vi "Super Market Billing System Final output.vi"() -> ()   [LabVIEW 2021]
uses:
  <vilib>/Utility/file.llb/Write Delimited Spreadsheet (string).vi
  <vilib>/regexp/Match Regular Expression.xnode
panel:
  in  "Tab Control":enum32{"Page 1", "Page 2", "Page 3"}(tab)
  out "Horizontal Progress Bar":u8(slide) scale=0.0..100.0
  in  "Password":string
  in  "Cashier User Name":string
  in  "OK Button":bool
  in  "Rice 5kg":bool
  in  "Dal 1kg":bool
  in  "Salt 400g":bool
  in  "Coconut Oil 1L":bool
  in  "Chilli Powder 100g":bool
  in  "Curry Powder 100g":bool
  in  "Turmeric Powder 50g":bool
  in  "Milk Powder 1kg":bool
  in  "Sugar  1kg":bool
  out "Rs.":dbl
  out "Rs.":dbl
  out "Rs.":dbl
  out "Rs.":dbl
  in  "Quantitiy":dbl min=0.0 format="%#.1f"
  out "Rs.":dbl
  in  "Quantitiy":dbl min=0.0 format="%#.1f"
  out "Rs":dbl
  in  "Quantitiy":dbl min=0.0 format="%#.1f"
  out "Rs.":dbl
  in  "Quantitiy":dbl min=0.0 format="%#.1f"
  in  "Quantitiy":dbl min=0.0 format="%#.1f"
  in  "Quantitiy":dbl min=0.0 format="%#.1f"
  in  "Quantitiy":dbl min=0.0 format="%#.1f"
  in  "Quantitiy":dbl min=0.0 format="%#.1f"
  in  "Tea 100g":bool
  in  "Quantitiy":dbl min=0.0 format="%#.1f"
  in  "Quantitiy":dbl min=0.0 format="%#.1f"
  out "Rs.":dbl
  out "Rs.":dbl
  out "Rs.":dbl
  out "Rs.":dbl
  out "Rs.":dbl
  out "Rs.":dbl
  out "Rs.":dbl
  out "Rs. 5":dbl
  out "Rs. 6":dbl
  out "Rs.":dbl
  out "Rs.":dbl
  out "Rs.":dbl
  out "Rs.":dbl
  out "Discount   Rs.":dbl format="%#.2f"
  in  "kg":dbl min=0.0 format="%#.3f"
  in  "Papaya":bool
  in  "kg":dbl min=0.0 format="%#.3f"
  in  "Graps":bool
  in  "kg":dbl min=0.0 format="%#.3f"
  in  "Orange":bool
  in  "kg":dbl min=0.0 format="%#.3f"
  in  "Apple":bool
  in  "kg":dbl min=0.0 format="%#.3f"
  in  "Banana":bool
  out "Bill   Rs.":dbl format="%#.2f"
  out "Discount percentage":string
  out "Total Bill   Rs.":dbl format="%#.2f"
  in  "kg":dbl min=0.0 format="%#.3f"
  in  "Cabege":bool
  in  "kg":dbl min=0.0 format="%#.3f"
  in  "Bringle":bool
  in  "kg":dbl min=0.0 format="%#.3f"
  in  "Beans":bool
  in  "kg":dbl min=0.0 format="%#.3f"
  in  "Leeks":bool
  in  "kg":dbl min=0.0 format="%#.3f"
  in  "Carrot":bool
  in  "stop":bool
  in  "stop 2":bool
  out "Bill Details":string
  in  "stop 3":bool
  # "WELCOME   TO  ABC                  SUPERMARCKET.."
  # "Price per 1kg (Rs.)"
  # "Quantities(kg)"
  # "Price  (Rs.)"
  # "Quantities"
  # "Fruits"
  # "Product List"
  # "Vegetables"
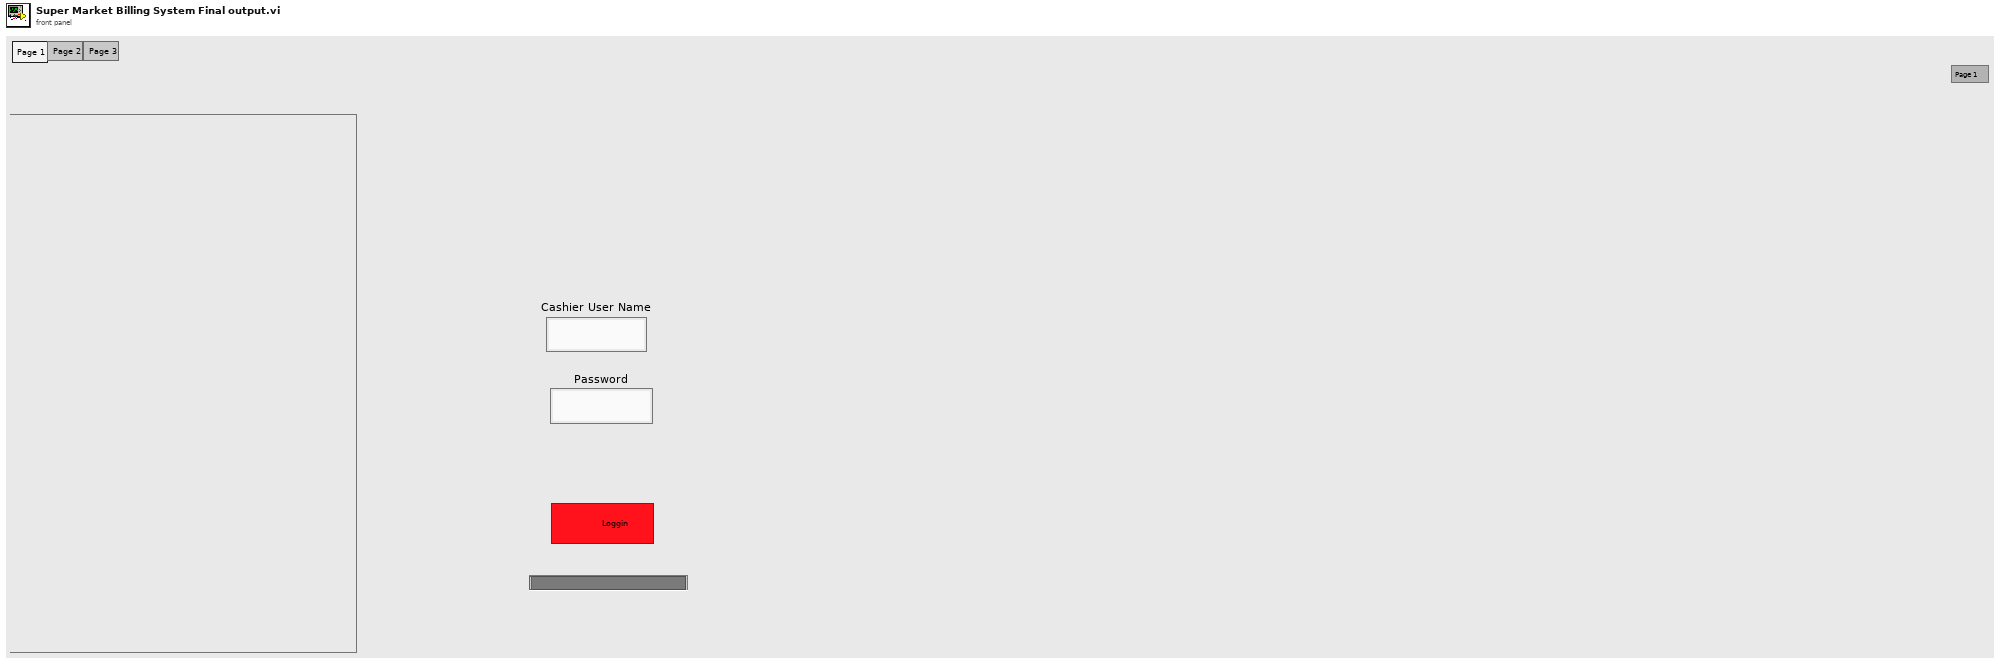
[diagram p1: front panel]
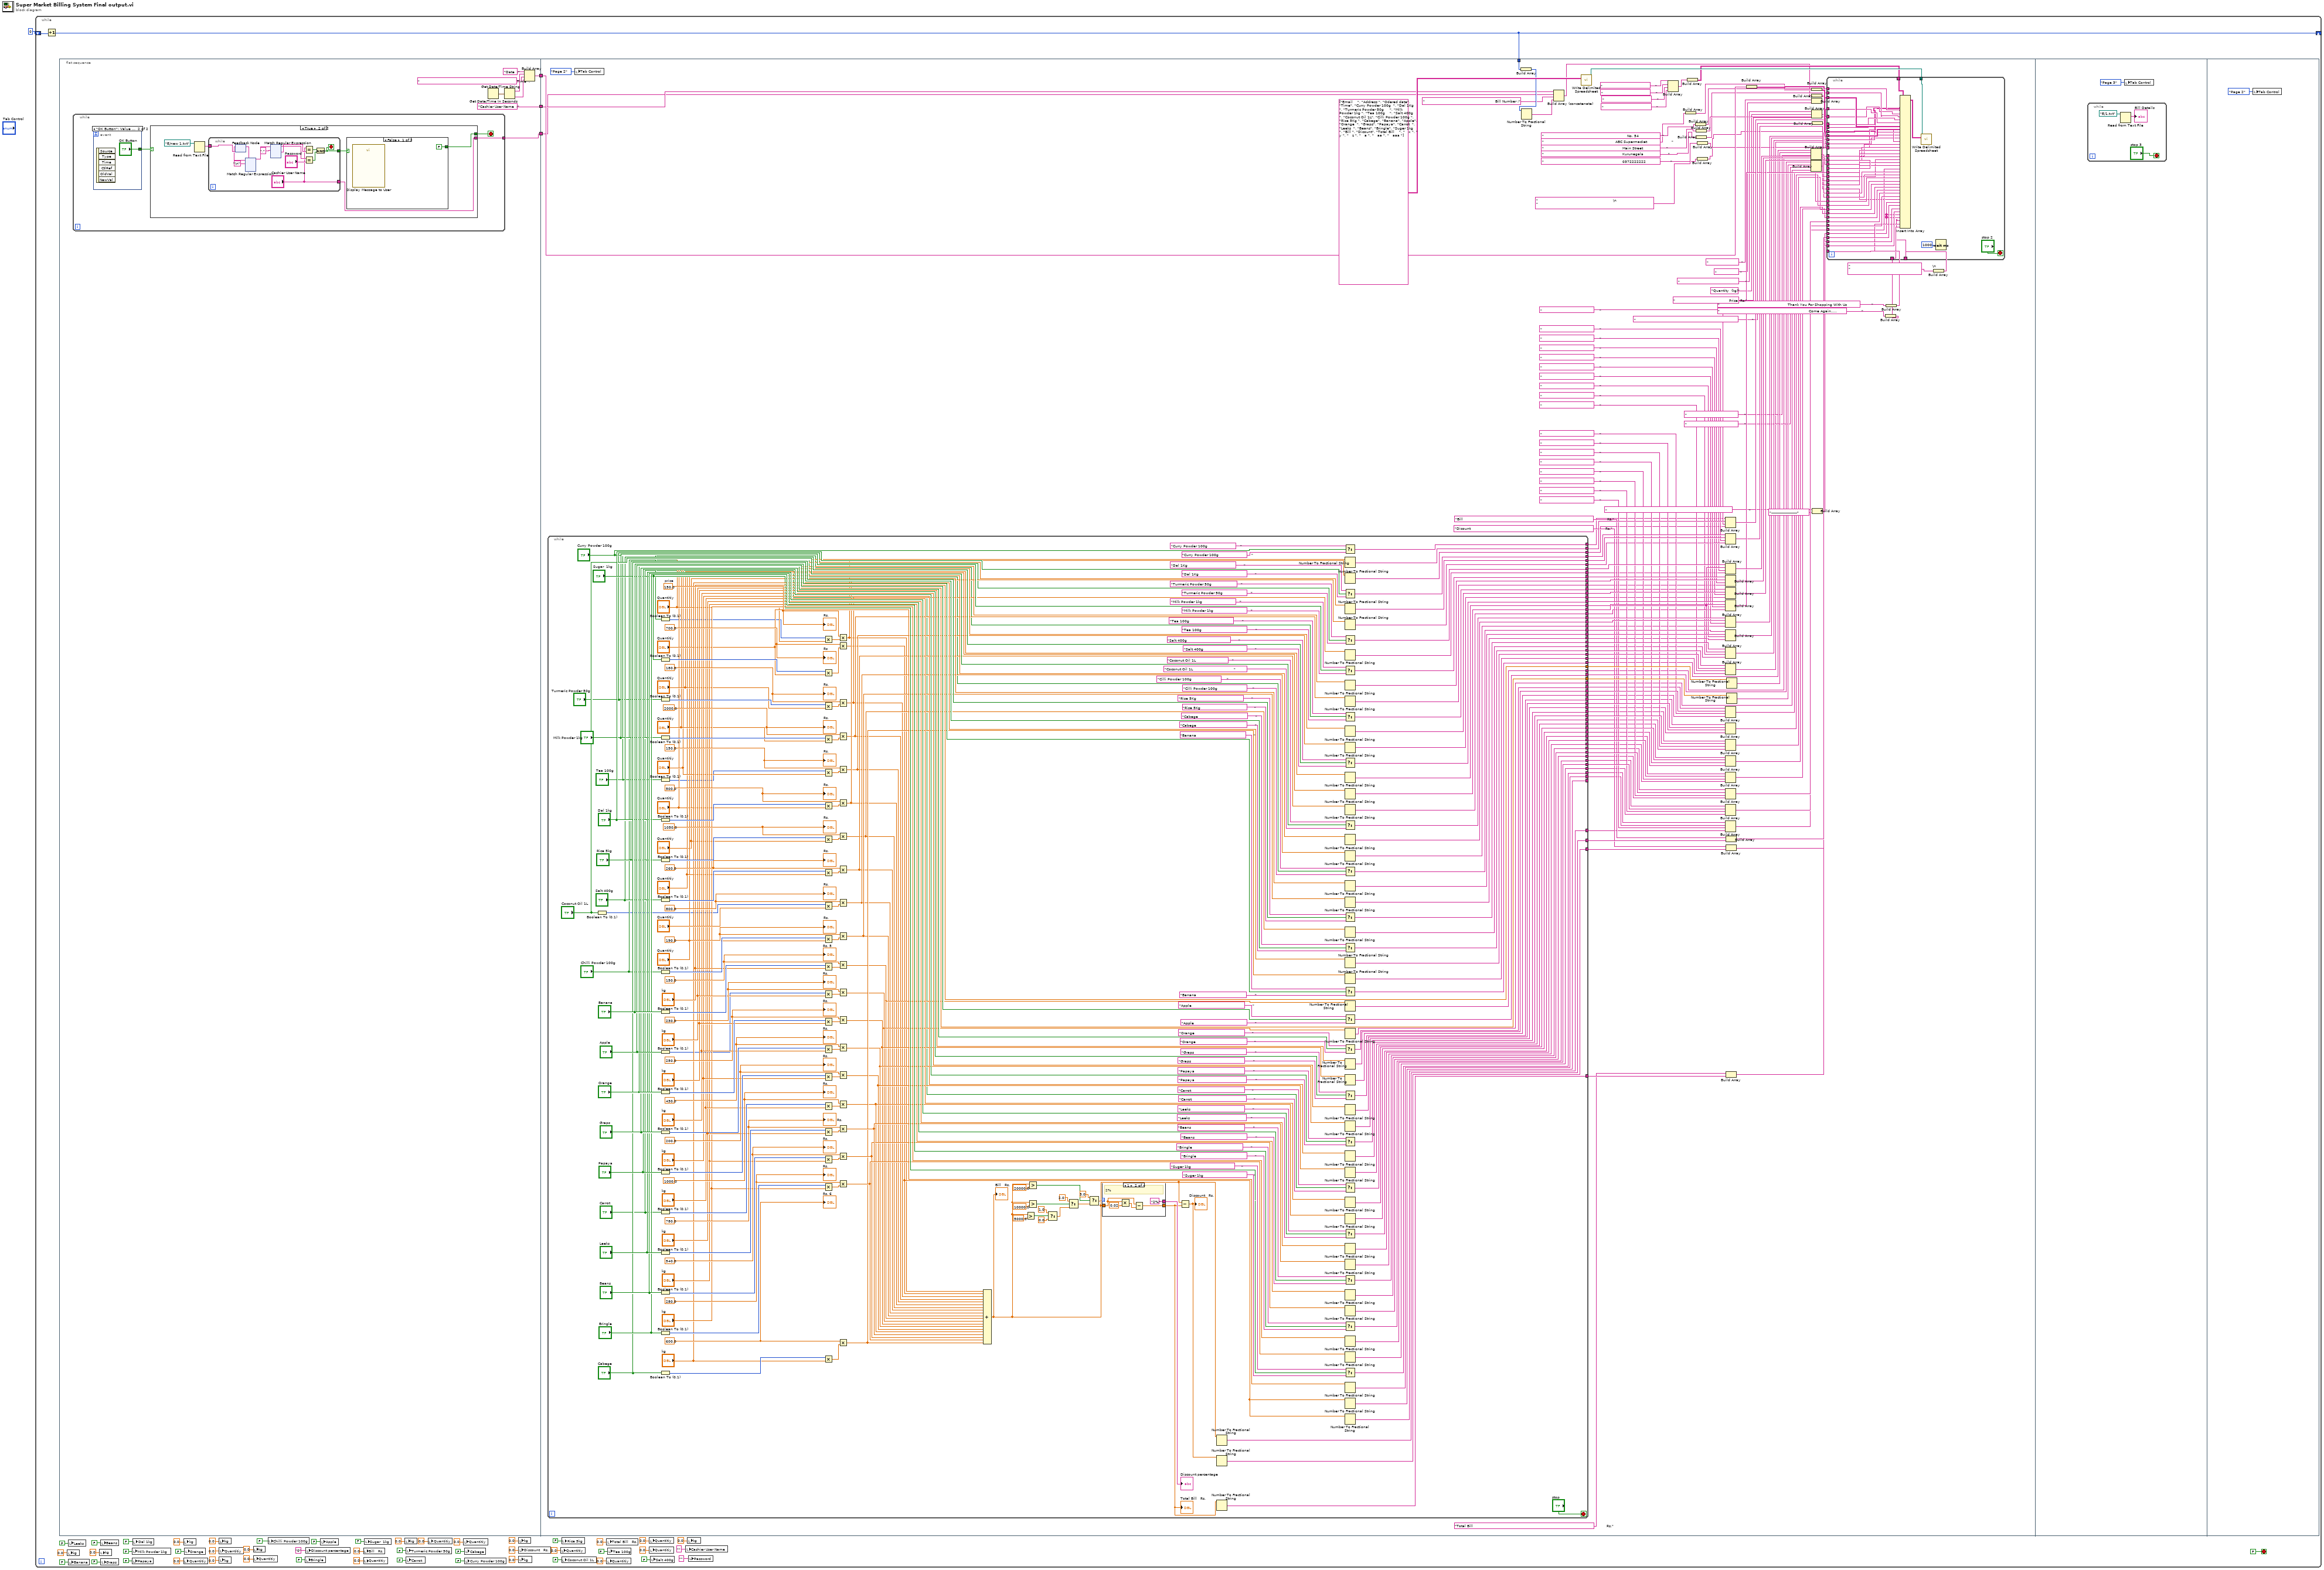
[diagram p0: block diagram]
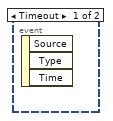
[diagram p2: hidden frame]
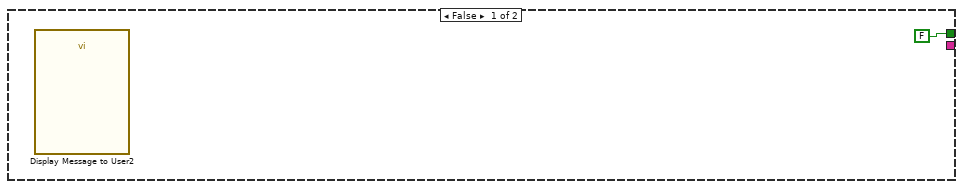
[diagram p3: hidden frame]
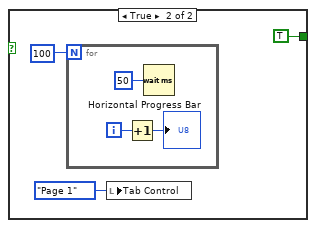
[diagram p4: hidden frame]
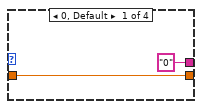
[diagram p5: hidden frame]
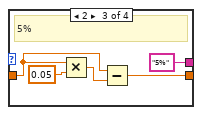
[diagram p6: hidden frame]
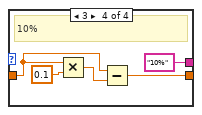
[diagram p7: hidden frame]
diagram:
  n1 = while {
    shift-right: [w4] -> _
    shift-left: 0 -> [w5]
    stop <- FALSE stop-if-true
    n2 = Increment(x=w5) -> (x+1=w4:i32)
    n3 = flat-sequence {
      tunnel: [w59] -> w53
      tunnel: ["Cashier User Name  :" ("element")] -> w3
      tunnel: [w54] -> w2
      tunnel: w53 -> [w363]
      tunnel: w4 -> [w332]
      tunnel: w3 -> [w330]
      tunnel: w2 -> [w329]
      frame #0 {
        n4 = while {
          tunnel: [w64] -> w54
          stop <- w63 stop-if-true
          n5 = event shown="[1] \"OK Button\": Value Change" {
            selector: _ -> [_ _]
            dyn-events: _ -> [_ _]
            timeout: _ -> [_ _]
            tunnel: [_ "OK Button"] -> w62
            event Timeout {
              n6 = event-data() -> ()  [unwired: 1 in, 3 out]
            }
            event "OK Button": Value Change {
              n7 = event-data() -> ()  [unwired: 1 in, 6 out]
            }
          }
          n8 = case shown="True" w62 {
            tunnel: [_ w69] -> w64
            tunnel: [FALSE w68] -> w63
            frame False {
              n9 = call "Display Message to User2"() -> ()  [unwired: 10 in, 2 out]
            }
            frame True {
              n10 = Read from Text File(file (use dialog)=path "E:/new 1.txt") -> (text=w71:string)  [unwired: 3 in, 3 out]
              n11 = while {
                tunnel: w71 -> [w91]
                tunnel: ["Cashier User Name"] -> w69
                tunnel: [w79] -> w67
                stop <- w79 stop-if-true
                n12 = feedback #1(w91) -> (w90:string)
                n13 = xnode "Match Regular Expression"("input string"=w90, "regular expression"="\n") -> ("before match"=w87:string, "after match"=w89:string)  [unwired: 4 in, 3 out]
                n14 = feedback-in #1(w89) -> ()
                n15 = xnode "Match Regular Expression"("input string"=w87, "regular expression"=",") -> ("before match"=w84:string, "after match"=w85:string)  [unwired: 4 in, 3 out]
                n16 = Equal?(x="Cashier User Name", y=w84) -> (x = y?=w82:bool)
                n17 = Equal?(x=w85, y="Password") -> (x = y?=w81:bool)
                n18 = And(x=w82, y=w81) -> (x .and. y?=w79:bool)
              }
              n19 = case shown="False" w67 {
                tunnel: [FALSE TRUE] -> w68
                frame False {
                  n20 = call "Display Message to User"() -> ()  [unwired: 10 in, 2 out]
                }
                frame True {
                  n21 = for {
                    N: 100 -> [_]
                    i -> [w76]
                    n22 = Increment(x=w76) -> (x+1=→"Horizontal Progress Bar":i32)
                    n23 = Wait (ms)(milliseconds to wait=u32 50 ("millisecond timer value")) -> ()  [unwired: 1 out]
                  }
                  n24 = local write "Tab Control"(enum32{"Page 1", "Page 2"}."Page 1" ("Tab Control")) -> ()
                }
              }
            }
          }
        }
        n25 = Get Date/Time In Seconds() -> (seconds since 1Jan1904=w60:timestamp)
        n26 = Get Date/Time String(seconds (now)=w60) -> (date string=w58:string, time string=w61:string)  [unwired: 2 in]
        n27 = Build Array("Date  :" ("element"), w58, "                                                                                   Time  :" ("element"), w61) -> (w59:string[])
      }
      frame #1 {
        n28 = while {
          tunnel: [w700] -> w480
          tunnel: [w697] -> w481
          tunnel: [w696] -> w482
          tunnel: [w688] -> w399
          tunnel: [w668] -> w451
          tunnel: [w667] -> w373
          tunnel: [w659] -> w369
          tunnel: [w658] -> w368
          tunnel: [w657] -> w367
          tunnel: [w656] -> w366
          tunnel: [w655] -> w370
          tunnel: [w654] -> w371
          tunnel: [w653] -> w442
          tunnel: ["kg"] -> w485
          tunnel: ["kg"] -> w484
          tunnel: [w649] -> w449
          tunnel: [w647] -> w448
          tunnel: [w644] -> w447
          tunnel: [w643] -> w446
          tunnel: [w642] -> w445
          tunnel: [w639] -> w444
          tunnel: [w636] -> w443
          tunnel: [w635] -> w441
          tunnel: [w608] -> w372
          tunnel: [w607] -> w345
          tunnel: [w606] -> w478
          tunnel: [w605] -> w477
          tunnel: [w604] -> w386
          tunnel: [w603] -> w474
          tunnel: [w602] -> w467
          tunnel: [w601] -> w471
          tunnel: [w600] -> w469
          tunnel: [w531] -> w468
          tunnel: [w597] -> w479
          tunnel: [w582] -> w419
          tunnel: [w595] -> w465
          tunnel: [w593] -> w476
          tunnel: [w591] -> w475
          tunnel: [w586] -> w473
          tunnel: [w529] -> w472
          tunnel: [w585] -> w470
          tunnel: [w584] -> w466
          tunnel: [w581] -> w418
          tunnel: [w580] -> w416
          tunnel: [w559] -> w414
          tunnel: [w558] -> w412
          tunnel: [w557] -> w410
          tunnel: [w555] -> w408
          tunnel: [w554] -> w406
          tunnel: [w543] -> w404
          tunnel: [w553] -> w402
          tunnel: [w552] -> w400
          tunnel: [w542] -> w397
          tunnel: [w551] -> w395
          tunnel: [w550] -> w392
          tunnel: [w549] -> w391
          tunnel: [w538] -> w389
          tunnel: [w548] -> w387
          tunnel: [w537] -> w384
          tunnel: [w547] -> w382
          tunnel: [w546] -> w380
          tunnel: [w545] -> w378
          tunnel: [w544] -> _
          stop <- "stop" stop-if-true
          w712 = 200.0 ("price")
          w709 = 430.0 ("price")
          w706 = 250.0 ("price")
          w704 = 230.0 ("price")
          w701 = 150.0 ("price")
          w727 = 600.0 ("price")
          w724 = 280.0 ("price")
          w721 = 540.0 ("price")
          w718 = 780.0 ("price")
          w715 = 1000.0 ("price")
          w754 = 150.0 ("price")
          w752 = 700.0 ("price")
          w749 = 2000.0 ("price")
          w746 = 180.0 ("price")
          w743 = 150.0  # price
          w766 = 190.0 ("price")
          w764 = 800.0 ("price")
          w761 = 260.0 ("price")
          w759 = 500.0 ("price")
          w756 = 1050.0 ("price")
          n29 = Boolean To (0,1)(Boolean="Coconut Oil 1L") -> (0, 1=w539:i16)
          n30 = Boolean To (0,1)(Boolean="Curry Powder 100g") -> (0, 1=w532:i16)
          n31 = Boolean To (0,1)(Boolean="Sugar  1kg") -> (0, 1=w753:i16)
          n32 = Boolean To (0,1)(Boolean="Turmeric Powder 50g") -> (0, 1=w747:i16)
          n33 = Boolean To (0,1)(Boolean="Milk Powder 1kg") -> (0, 1=w748:i16)
          n34 = Boolean To (0,1)(Boolean="Tea 100g") -> (0, 1=w535:i16)
          n35 = Boolean To (0,1)(Boolean="Dal 1kg") -> (0, 1=w693:i16)
          n36 = Boolean To (0,1)(Boolean="Rice 5kg") -> (0, 1=w695:i16)
          n37 = Boolean To (0,1)(Boolean="Salt 400g") -> (0, 1=w760:i16)
          n38 = Boolean To (0,1)(Boolean="Chilli Powder 100g") -> (0, 1=w694:i16)
          n39 = Boolean To (0,1)(Boolean="Banana") -> (0, 1=w692:i16)
          n40 = Boolean To (0,1)(Boolean="Apple") -> (0, 1=w541:i16)
          n41 = Boolean To (0,1)(Boolean="Orange") -> (0, 1=w705:i16)
          n42 = Boolean To (0,1)(Boolean="Graps") -> (0, 1=w710:i16)
          n43 = Boolean To (0,1)(Boolean="Papaya") -> (0, 1=w711:i16)
          n44 = Boolean To (0,1)(Boolean="Carrot") -> (0, 1=w714:i16)
          n45 = Boolean To (0,1)(Boolean="Leeks") -> (0, 1=w719:i16)
          n46 = Boolean To (0,1)(Boolean="Beans") -> (0, 1=w720:i16)
          n47 = Boolean To (0,1)(Boolean="Bringle") -> (0, 1=w725:i16)
          n48 = Boolean To (0,1)(Boolean="Cabege") -> (0, 1=w726:i16)
          n49 = Multiply(x=w532, y="Quantitiy") -> (x*y=w744:dbl)
          n50 = Multiply(x=w753, y="Quantitiy") -> (x*y=w751:dbl)
          n51 = Multiply(x=w747, y="Quantitiy") -> (x*y=w745:dbl)
          n52 = Multiply(x=w748, y="Quantitiy") -> (x*y=w750:dbl)
          n53 = Multiply(x=w535, y="Quantitiy") -> (x*y=w755:dbl)
          n54 = Multiply(x=w693, y="Quantitiy") -> (x*y=w758:dbl)
          n55 = Multiply(x=w695, y="Quantitiy") -> (x*y=w757:dbl)
          n56 = Multiply(x=w760, y="Quantitiy") -> (x*y=w762:dbl)
          n57 = Multiply(x=w539, y="Quantitiy") -> (x*y=w763:dbl)
          n58 = Multiply(x=w694, y="Quantitiy") -> (x*y=w767:dbl)
          n59 = Multiply(x=w692, y="kg") -> (x*y=w702:dbl)
          n60 = Multiply(x=w541, y="kg") -> (x*y=w703:dbl)
          n61 = Multiply(x=w705, y="kg") -> (x*y=w707:dbl)
          n62 = Multiply(x=w710, y="kg") -> (x*y=w708:dbl)
          n63 = Multiply(x=w711, y="kg") -> (x*y=w713:dbl)
          n64 = Multiply(x=w714, y="kg") -> (x*y=w716:dbl)
          n65 = Multiply(x=w719, y="kg") -> (x*y=w717:dbl)
          n66 = Multiply(x=w720, y="kg") -> (x*y=w722:dbl)
          n67 = Multiply(x=w725, y="kg") -> (x*y=w723:dbl)
          n68 = Multiply(x=w726, y="kg") -> (x*y=w728:dbl)
          n69 = Multiply(x=w743, y=w744) -> (x*y=w533:dbl)
          n70 = Multiply(x=w752, y=w751) -> (x*y=w560:dbl)
          n71 = Multiply(x=w746, y=w745) -> (x*y=w562:dbl)
          n72 = Multiply(x=w749, y=w750) -> (x*y=w563:dbl)
          n73 = Multiply(x=w754, y=w755) -> (x*y=w564:dbl)
          n74 = Multiply(x=w759, y=w758) -> (x*y=w566:dbl)
          n75 = Multiply(x=w756, y=w757) -> (x*y=w565:dbl)
          n76 = Multiply(x=w761, y=w762) -> (x*y=w567:dbl)
          n77 = Multiply(x=w764, y=w763) -> (x*y=w568:dbl)
          n78 = Multiply(x=w766, y=w767) -> (x*y=w569:dbl)
          n79 = Multiply(x=w701, y=w702) -> (x*y=w570:dbl)
          n80 = Multiply(x=w704, y=w703) -> (x*y=w571:dbl)
          n81 = Multiply(x=w706, y=w707) -> (x*y=w572:dbl)
          n82 = Multiply(x=w709, y=w708) -> (x*y=w573:dbl)
          n83 = Multiply(x=w712, y=w713) -> (x*y=w574:dbl)
          n84 = Multiply(x=w715, y=w716) -> (x*y=w575:dbl)
          n85 = Multiply(x=w718, y=w717) -> (x*y=w578:dbl)
          n86 = Multiply(x=w721, y=w722) -> (x*y=w577:dbl)
          n87 = Multiply(x=w724, y=w723) -> (x*y=w579:dbl)
          n88 = Multiply(x=w727, y=w728) -> (x*y=w576:dbl)
          n89 = Compound Arithmetic op=ADD(w533, w560, w562, w563, w564, w566, w565, w567, w568, w569, w570, w571, w572, w573, w574, w575, w578, w577, w579, w576) -> (w561:dbl)
          "Bill   Rs." <- w561
          n90 = Greater?(x=w561, y=5000.0) -> (0:w740:bool)
          n91 = Greater?(x=w561, y=20000.0) -> (0:w742:bool)
          n92 = Greater?(x=w561, y=10000.0) -> (0:w741:bool)
          n93 = Select(t=1.0, s=w740, f=0.0) -> (s? t:f=w736:dbl)
          n94 = Select(t=2.0, s=w741, f=w736) -> (s? t:f=w737:dbl)
          n95 = Select(t=3.0, s=w742, f=w737) -> (s? t:f=w738:dbl)
          n96 = case shown="1" w738 {
            tunnel: [w769 w773 w776 w781] -> w699
            tunnel: w561 -> [w769 w772 w777 w782]
            tunnel: ["0" ("discount") "2%" ("discount") "5%" ("discount") "10%" ("discount")] -> w739
            frame 0, Default {
            }
            frame 1 {
              # "2%"
              n97 = Multiply(x=w772, y=0.02) -> (x*y=w770:dbl)
              n98 = Subtract(x=w772, y=w770) -> (x-y=w773:dbl)
            }
            frame 2 {
              # "5%"
              n99 = Multiply(x=w777, y=0.05) -> (x*y=w778:dbl)
              n100 = Subtract(x=w777, y=w778) -> (x-y=w776:dbl)
            }
            frame 3 {
              # "10%"
              n101 = Multiply(x=w782, y=0.1) -> (x*y=w783:dbl)
              n102 = Subtract(x=w782, y=w783) -> (x-y=w781:dbl)
            }
          }
          "Total Bill   Rs." <- w699
          "Discount percentage" <- w739
          n103 = Subtract(x=w561, y=w699) -> (x-y=w698:dbl)
          "Discount   Rs." <- w698
          n104 = Number To Fractional String(number=w561) -> (F-format string=w700:string)  [unwired: 3 in]
          n105 = Number To Fractional String(number=w698) -> (F-format string=w696:string)  [unwired: 3 in]
          n106 = Number To Fractional String(number=w699) -> (F-format string=w697:string)  [unwired: 3 in]
          n107 = Select(t="Curry Powder 100g                            ", s="Curry Powder 100g", f="Curry Powder 100g                            ") -> (s? t:f=w607:string)
          n108 = Number To Fractional String(number="Quantitiy") -> (F-format string=w597:string)  [unwired: 3 in]
          n109 = Number To Fractional String(number=w533) -> (F-format string=w545:string)  [unwired: 3 in]
          n110 = Select(t="Dal 1Kg                                                ", s="Dal 1kg", f="Dal 1Kg                                                ") -> (s? t:f=w531:string)
          n111 = Number To Fractional String(number="Quantitiy") -> (F-format string=w584:string)  [unwired: 3 in]
          n112 = Number To Fractional String(number=w566) -> (F-format string=w538:string)  [unwired: 3 in]
          n113 = Select(t="Turmeric Powder 50g                         ", s="Turmeric Powder 50g", f="Turmeric Powder 50g                        ") -> (s? t:f=w606:string)
          n114 = Number To Fractional String(number=w562) -> (F-format string=w546:string)  [unwired: 3 in]
          n115 = Select(t="Milk Powder 1kg                                ", s="Milk Powder 1kg", f="Milk Powder 1kg                                ") -> (s? t:f=w605:string)
          n116 = Number To Fractional String(number="Quantitiy") -> (F-format string=w593:string)  [unwired: 3 in]
          n117 = Number To Fractional String(number=w563) -> (F-format string=w547:string)  [unwired: 3 in]
          n118 = Select(t="Tea 100g                                             ", s="Tea 100g", f="Tea 100g                                              ") -> (s? t:f=w604:string)
          n119 = Number To Fractional String(number="Quantitiy") -> (F-format string=w591:string)  [unwired: 3 in]
          n120 = Number To Fractional String(number=w564) -> (F-format string=w537:string)  [unwired: 3 in]
          n121 = Select(t="Salt 400g                                            ", s="Salt 400g", f="Salt 400g                                            ") -> (s? t:f=w603:string)
          n122 = Number To Fractional String(number="Quantitiy") -> (F-format string=w595:string)  [unwired: 3 in]
          n123 = Number To Fractional String(number="Quantitiy") -> (F-format string=w586:string)  [unwired: 3 in]
          n124 = Number To Fractional String(number=w567) -> (F-format string=w549:string)  [unwired: 3 in]
          n125 = Select(t="Coconut Oil 1L                               ", s="Coconut Oil 1L", f="Coconut Oil 1L                                   ") -> (s? t:f=w602:string)
          n126 = Number To Fractional String(number="Quantitiy") -> (F-format string=w529:string)  [unwired: 3 in]
          n127 = Number To Fractional String(number=w568) -> (F-format string=w550:string)  [unwired: 3 in]
          n128 = Select(t="Cilli Powder 100g                              ", s="Chilli Powder 100g", f="Cilli Powder 100g                              ") -> (s? t:f=w601:string)
          n129 = Number To Fractional String(number="Quantitiy") -> (F-format string=w585:string)  [unwired: 3 in]
          n130 = Number To Fractional String(number=w569) -> (F-format string=w551:string)  [unwired: 3 in]
          n131 = Select(t="Rise 5Kg                                               ", s="Rice 5kg", f="Rise 5Kg                                              ") -> (s? t:f=w600:string)
          n132 = Number To Fractional String(number=w565) -> (F-format string=w548:string)  [unwired: 3 in]
          n133 = Select(t="Cabege                                                 ", s="Cabege", f="Cabege                                                  ") -> (s? t:f=w653:string)
          n134 = Number To Fractional String(number="kg") -> (F-format string=w635:string)  [unwired: 3 in]
          n135 = Number To Fractional String(number=w576) -> (F-format string=w559:string)  [unwired: 3 in]
          n136 = Select(t="Banana                                                 ", s="Banana", f="Banana                                                  ") -> (s? t:f=w688:string)
          n137 = Number To Fractional String(number=w570) -> (F-format string=w542:string)  [unwired: 3 in]
          n138 = Select(t="Apple                                                    ", s="Apple", f="Apple                                                    ") -> (s? t:f=w668:string)
          n139 = Number To Fractional String(number=w571) -> (F-format string=w552:string)  [unwired: 3 in]
          n140 = Select(t="Orange                                                 ", s="Orange", f="Orange                                                  ") -> (s? t:f=w667:string)
          n141 = Number To Fractional String(number="kg") -> (F-format string=w649:string)  [unwired: 3 in]
          n142 = Number To Fractional String(number=w572) -> (F-format string=w553:string)  [unwired: 3 in]
          n143 = Select(t="Graps                                                    " ("f"), s="Graps", f="Graps                                                     ") -> (s? t:f=w659:string)
          n144 = Number To Fractional String(number="kg") -> (F-format string=w647:string)  [unwired: 3 in]
          n145 = Number To Fractional String(number=w573) -> (F-format string=w543:string)  [unwired: 3 in]
          n146 = Select(t="Papaya                                                  ", s="Papaya", f="Papaya                                                    ") -> (s? t:f=w658:string)
          n147 = Number To Fractional String(number="kg") -> (F-format string=w644:string)  [unwired: 3 in]
          n148 = Number To Fractional String(number=w574) -> (F-format string=w554:string)  [unwired: 3 in]
          n149 = Select(t="Carrot                                                    ", s="Carrot", f="Carrot                                                     ") -> (s? t:f=w657:string)
          n150 = Number To Fractional String(number="kg") -> (F-format string=w643:string)  [unwired: 3 in]
          n151 = Number To Fractional String(number=w575) -> (F-format string=w555:string)  [unwired: 3 in]
          n152 = Select(t="Leeks                                                     ", s="Leeks", f="Leeks                                                    ") -> (s? t:f=w656:string)
          n153 = Number To Fractional String(number="kg") -> (F-format string=w642:string)  [unwired: 3 in]
          n154 = Number To Fractional String(number=w578) -> (F-format string=w557:string)  [unwired: 3 in]
          n155 = Select(t="Beans                                                     ", s="Beans", f="Beans                                                    ") -> (s? t:f=w655:string)
          n156 = Number To Fractional String(number="kg") -> (F-format string=w639:string)  [unwired: 3 in]
          n157 = Number To Fractional String(number=w577) -> (F-format string=w558:string)  [unwired: 3 in]
          n158 = Select(t="Bringle                                                  ", s="Bringle", f="Bringle                                                  ") -> (s? t:f=w654:string)
          n159 = Number To Fractional String(number="kg") -> (F-format string=w636:string)  [unwired: 3 in]
          n160 = Number To Fractional String(number=w579) -> (F-format string=w580:string)  [unwired: 3 in]
          n161 = Select(t="Suger 1kg                                           ", s="Sugar  1kg", f="Suger 1kg                                           ") -> (s? t:f=w608:string)
          n162 = Number To Fractional String(number="Quantitiy") -> (F-format string=w582:string)  [unwired: 3 in]
          n163 = Number To Fractional String(number=w560) -> (F-format string=w544:string)  [unwired: 3 in]
          n164 = Number To Fractional String(number=w560) -> (F-format string=w581:string)  [unwired: 3 in]
          "Rs." <- w756
          "Rs." <- w759
          "Rs." <- w761
          "Rs." <- w764
          "Rs." <- w766
          "Rs." <- w743
          "Rs." <- w746
          "Rs." <- w749
          "Rs" <- w752
          "Rs." <- w754
          "Rs." <- w715
          "Rs." <- w718
          "Rs." <- w721
          "Rs." <- w724
          "Rs. 6" <- w727
          "Rs. 5" <- w701
          "Rs." <- w704
          "Rs." <- w706
          "Rs." <- w709
          "Rs." <- w712
        }
        n165 = local write "Tab Control"(enum32{"Page 1", "Page 2"}."Page 2" ("Tab Control")) -> ()
        n166 = Build Array(w332) -> (w331:i32[])
        n167 = Number To Fractional String(number=w331) -> (F-format string=w326:string[])  [unwired: 3 in]
        n168 = Build Array (concatenate)(w330, w329, "                                                            Bill Number :", w326) -> (w328:string[])
        n169 = call-poly <vilib>:"Write Delimited Spreadsheet.vi"("2D data"=string[][] [["Email    "], ["Address "], ["Odered date"], ["Time"], ["Curry Powder 100g  "], ["Dal 1Kg   "], ["Turmeric Powder 50g     "], ["Milk Powder 1kg "], ["Tea 100g    "], ["Salt 400g   "], ["Coconut Oil 1L"], ["Cilli Powder 100g "], ["Rise 5Kg "], ["Cabege"], ["Banana"], ["Apple"], ["Orange  "], ["Graps"], ["Papaya"], ["Carrot  "], ["Leeks  "], ["Beans"], ["Bringle"], ["Suger 1kg  "], ["Bill "], ["Dicount"], ["Total Bill    "], ["   x "], ["   y "], ["   z "], ["   a "], ["   aa "], ["   aaa "]] ("delimiter (\\t)")) -> ("new file path (Not A Path if cancelled)"=w364:path)  [unwired: 13 in, 1 out]
        n170 = Build Array("                                             ", "                                             ", "                                             ", "                                             ") -> (w354:string[])
        n171 = Build Array("                                                             ABC Supermacket                     ") -> (w341:string[])
        n172 = Build Array(w354) -> (w349:string[][])
        n173 = Build Array("                                                                       No. 54                    ") -> (w358:string[])
        n174 = Build Array("                                                                   Main Street                    ") -> (w357:string[])
        n175 = Build Array("                                                                   Kurunegala                     ") -> (w356:string[])
        n176 = Build Array("                                                                   0372222222                     ") -> (w339:string[])
        n177 = Build Array("                                                                \n                                                ") -> (w355:string[])
        n178 = Build Array(w345, w479, "                                                 " ("element"), w378) -> (w461:string[])
        n179 = Build Array(w468, w466, "                                                 " ("element"), w389) -> (w453:string[])
        n180 = Build Array(w478, w465, "                                                 " ("element"), w380) -> (w460:string[])
        n181 = Build Array(w477, w476, "                                                 " ("element"), w382) -> (w459:string[])
        n182 = Build Array(w386, w475, "                                                 " ("element"), w384) -> (w458:string[])
        n183 = Build Array(w474, w473, "                                                 " ("element"), w391) -> (w457:string[])
        n184 = Build Array(w467, w472, "                                                 " ("element"), w392) -> (w456:string[])
        n185 = Build Array(w471, w470, "                                                 " ("element"), w395) -> (w455:string[])
        n186 = Build Array(w469, w465, "                                                 " ("element"), w387) -> (w454:string[])
        n187 = Build Array(w442, w441, "                                                 " ("element"), w414) -> (w333:string[])
        n188 = Build Array(w373, w449, "                                                 " ("element"), w402) -> (w438:string[])
        n189 = Build Array(w369, w448, "                                                 " ("element"), w404) -> (w437:string[])
        n190 = Build Array(w368, w447, "                                                 " ("element"), w406) -> (w436:string[])
        n191 = Build Array(w367, w446, "                                                 " ("element"), w408) -> (w435:string[])
        n192 = Build Array(w366, w445, "                                                 " ("element"), w410) -> (w434:string[])
        n193 = Build Array(w370, w444, "                                                 " ("element"), w412) -> (w433:string[])
        n194 = Build Array(w371, w443, "                                                 " ("element"), w416) -> (w432:string[])
        n195 = Build Array(w372, w419, "                                                 " ("element"), w418) -> (w334:string[])
        n196 = Build Array("Bill                                                                                                                           Rs." ("element"), w480) -> (w463:string[])
        n197 = Build Array("Dicount                                                                                                                   Rs." ("element"), w482) -> (w421:string[])
        n198 = Build Array("Total Bill                                                                                                                  Rs." ("element"), w481) -> (w462:string[])
        n199 = Number To Fractional String(number=w485) -> (F-format string=w452:string)  [unwired: 3 in]
        n200 = Number To Fractional String(number=w484) -> (F-format string=w450:string)  [unwired: 3 in]
        n201 = Build Array(w363) -> (w362:string[][])
        n202 = Build Array(w399, w452, "                                                 " ("element"), w397) -> (w440:string[])
        n203 = Build Array(w451, w450, "                                                 " ("element"), w400) -> (w439:string[])
        n204 = Build Array("                                                        " ("element"), "Quantity  (kg)" ("element"), "                                              Price  Rs." ("element")) -> (w423:string[])
        n205 = Build Array(w341) -> (w464:string[][])
        n206 = Build Array(w328) -> (w429:string[][])
        n207 = Build Array("                            ", "                    " ("element")) -> (w425:string[])
        n208 = Build Array("                                                                                                   ") -> (w344:string[])
        n209 = Build Array("                                                                                                                         ", "----------------------" ("element")) -> (w376:string[])
        n210 = Build Array("                                                                            Come Again.....                     " ("element")) -> (w337:string[])
        n211 = Build Array("                                                          Thank You For Shopping With Us                     " ("element")) -> (w343:string[])
        n212 = Build Array("                                                                      \n                                                     " ("element")) -> (w335:string[])
        n213 = while {
          tunnel: w364 -> [w528]
          tunnel: w464 -> [w486]
          tunnel: w463 -> [w507]
          tunnel: w421 -> [w506]
          tunnel: w462 -> [w505]
          tunnel: w334 -> [w494]
          tunnel: w461 -> [w501]
          tunnel: w460 -> [w510]
          tunnel: w459 -> [w511]
          tunnel: w458 -> [w512]
          tunnel: w457 -> [w513]
          tunnel: w456 -> [w514]
          tunnel: w455 -> [w515]
          tunnel: w454 -> [w516]
          tunnel: w453 -> [w509]
          tunnel: w440 -> [w517]
          tunnel: w439 -> [w518]
          tunnel: w438 -> [w519]
          tunnel: w437 -> [w520]
          tunnel: w436 -> [w521]
          tunnel: w435 -> [w522]
          tunnel: w434 -> [w523]
          tunnel: w433 -> [w524]
          tunnel: w432 -> [w525]
          tunnel: w333 -> [w493]
          tunnel: w429 -> [w526]
          tunnel: w425 -> [w508]
          tunnel: w423 -> [w500]
          tunnel: w376 -> [w495]
          tunnel: w362 -> [w503]
          tunnel: w358 -> [w487]
          tunnel: w357 -> [w488]
          tunnel: w356 -> [w489]
          tunnel: w355 -> [w491]
          tunnel: w349 -> [w502]
          tunnel: w344 -> [w499]
          tunnel: w343 -> [w497]
          tunnel: w339 -> [w490]
          tunnel: w337 -> [w498]
          tunnel: w335 -> [w496]
          stop <- "stop 2" stop-if-true
          n214 = Insert Into Array(array=w502, new element #1=w486, new element #2=w487, new element #3=w488, new element #4=w489, new element #5=w490, new element #6=w491, new element #7=w503, new element #8=w526, new element #9=w508, new element #10=w499, new element #11=w500, new element #12=w501, new element #13=w509, new element #14=w510, new element #15=w511, new element #16=w512, new element #17=w513, new element #18=w514, new element #19=w515, new element #20=w516, new element #21=w494, new element #22=w517, new element #23=w518, new element #24=w519, new element #25=w520, new element #26=w521, new element #27=w522, new element #28=w523, new element #29=w524, new element #30=w525, new element #31=w493, new element #32=w495, new element #33=w507, new element #34=w506, new element #35=w505, new element #36=w495, new element #37=w495, new element #38=w496, new element #39=w497, new element #40=w498) -> (w504:string[][])  [unwired: 2 in]
          n215 = call-poly <vilib>:"Write Delimited Spreadsheet.vi"("file path (dialog if empty)"=w528, "2D data"=w504) -> ()  [unwired: 12 in, 2 out]
          n216 = Wait (ms)(milliseconds to wait=u32 1000) -> ()  [unwired: 1 out]
        }
      }
      frame #2 {
        n217 = while {
          stop <- "stop 3" stop-if-true
          n218 = Read from Text File(file (use dialog)=path "E:/1.txt") -> (text=→"Bill Details":string)  [unwired: 3 in, 3 out]
        }
        n219 = local write "Tab Control"(enum32{"Page 1", "Page 2", "Page 3"}."Page 3" ("Tab Control")) -> ()
      }
      frame #3 {
        n220 = local write "Tab Control"(enum32{"Page 1", "Page 2", "Page 3"}."Page 2" ("Tab Control")) -> ()
      }
    }
    n221 = local write "kg"(0.0 ("kg")) -> ()
    n222 = local write "Leeks"(FALSE ("Leeks")) -> ()
    n223 = local write "Banana"(FALSE ("Banana")) -> ()
    n224 = local write "kg"(0.0 ("kg")) -> ()
    n225 = local write "Beans"(FALSE ("Beans")) -> ()
    n226 = local write "Graps"(FALSE ("Graps")) -> ()
    n227 = local write "Milk Powder 1kg"(FALSE ("Milk Powder 1kg")) -> ()
    n228 = local write "Papaya"(FALSE ("Papaya")) -> ()
    n229 = local write "Dal 1kg"(FALSE ("Dal 1Kg")) -> ()
    n230 = local write "kg"(0.0 ("kg")) -> ()
    n231 = local write "Quantitiy"(0.0 ("Quantities")) -> ()
    n232 = local write "Orange"(FALSE ("Orange")) -> ()
    n233 = local write "kg"(0.0 ("kg")) -> ()
    n234 = local write "Quantitiy"(0.0 ("quantity 15")) -> ()
    n235 = local write "kg"(0.0 ("kg")) -> ()
    n236 = local write "kg"(0.0 ("kg")) -> ()
    n237 = local write "Quantitiy"(0.0 ("quantity 17")) -> ()
    n238 = local write "Chilli Powder 100g"(FALSE ("Cilli Powder 100g")) -> ()
    n239 = local write "Bringle"(FALSE ("Bringle")) -> ()
    n240 = local write "Discount percentage"("0" ("Discount percentage")) -> ()
    n241 = local write "Apple"(FALSE ("Apple")) -> ()
    n242 = local write "Bill   Rs."(0.0 ("Bill   Rs.")) -> ()
    n243 = local write "Quantitiy"(0.0 ("quantity 10")) -> ()
    n244 = local write "Sugar  1kg"(FALSE ("Sugar  1kg")) -> ()
    n245 = local write "kg"(0.0 ("kg")) -> ()
    n246 = local write "Turmeric Powder 50g"(FALSE ("Turmeric Powder 50g")) -> ()
    n247 = local write "Carrot"(FALSE ("Carrot")) -> ()
    n248 = local write "Quantitiy"(0.0 ("quantity 16")) -> ()
    n249 = local write "Quantitiy"(0.0 ("quantity 12")) -> ()
    n250 = local write "Cabege"(FALSE ("Cabege")) -> ()
    n251 = local write "Curry Powder 100g"(FALSE ("Curry Powder 100g")) -> ()
    n252 = local write "kg"(0.0 ("kg")) -> ()
    n253 = local write "Discount   Rs."(0.0 ("Discount   Rs.")) -> ()
    n254 = local write "kg"(0.0 ("kg")) -> ()
    n255 = local write "Quantitiy"(0.0 ("quantity 13")) -> ()
    n256 = local write "Rice 5kg"(FALSE ("Rise 5Kg")) -> ()
    n257 = local write "Coconut Oil 1L"(FALSE ("Coconut Oil 1L")) -> ()
    n258 = local write "Total Bill   Rs."(0.0 ("Total Bill   Rs.")) -> ()
    n259 = local write "Quantitiy"(0.0 ("quantity 14")) -> ()
    n260 = local write "Tea 100g"(FALSE ("Tea 100g")) -> ()
    n261 = local write "Quantitiy"(0.0 ("quantity 11")) -> ()
    n262 = local write "Quantitiy"(0.0 ("Quantities 4")) -> ()
    n263 = local write "Salt 400g"(FALSE ("Salt 400g")) -> ()
    n264 = local write "Cashier User Name"("" ("String")) -> ()
    n265 = local write "kg"(0.0 ("kg")) -> ()
    n266 = local write "Password"("" ("String 2")) -> ()
  }
